vi "Dresden R2R Sputter 03.02.2018 IY24.vi"() -> ()   [LabVIEW 2009] (continued)
                    n17084 = local read "Semi"() -> (w25564:bool)
                    n17085 = case shown="False" w25564 {
                      frame #0 {
                        n17086 = stacked-sequence {
                          frame #0 {
                            n17087 = local read "Semi"() -> (w25565:bool)
                            n17088 = case shown="False" w25565 {
                              frame #0 {
                                n17089 = while {
                                i -> [w25572]
                                stop <- w25568 stop-if-true
                                n17090 = Greater?(x=w25572, y=50) -> (0:w25566:bool)
                                n17091 = case shown="True" w25566 {
                                frame #0 {
                                }
                                frame #1 {
                                n17092 = local write "Error Message"("Start up process cancelled because\nthere is no enough air pressure.\nPlease check air pressure connections." ("Error Message")) -> ()
                                n17093 = local write "Semi"(TRUE ("Semi")) -> ()
                                }
                                }
                                n17094 = local read "Ch2_Air_press_di"() -> (w25567:bool)
                                n17095 = case shown="True" w25567 {
                                tunnel: [TRUE FALSE] -> w25570
                                frame #0 {
                                }
                                frame #1 {
                                n17096 = Wait Until Next ms Multiple(millisecond multiple=u32 200) -> ()  [unwired: 1 out]
                                }
                                }
                                n17097 = local read "Semi"() -> (w25569:bool)
                                n17098 = Or(x=w25570, y=w25569) -> (x .or. y?=w25568:bool)
                                }
                              }
                              frame #1 {
                              }
                            }
                          }
                          frame #1 {
                            n17099 = local read "Semi"() -> (w25578:bool)
                            n17100 = case shown="False" w25578 {
                              frame #0 {
                                n17101 = Wait Until Next ms Multiple(millisecond multiple=u32 1000) -> ()  [unwired: 1 out]
                                n17102 = local write "Ch2_PV0"(TRUE ("PA0")) -> ()
                                n17103 = local write "Ch2_PA0"(TRUE ("PA0")) -> ()
                              }
                              frame #1 {
                              }
                            }
                          }
                        }
                      }
                      frame #1 {
                      }
                    }
                  }
                  frame #2 {
                    n17104 = local read "Semi"() -> (w25582:bool)
                    n17105 = case shown="False" w25582 {
                      frame #0 {
                        n17106 = stacked-sequence {
                          frame #0 {
                            n17107 = local read "Semi"() -> (w25583:bool)
                            n17108 = case shown="False" w25583 {
                              frame #0 {
                                n17109 = while {
                                i -> [w25590]
                                stop <- w25586 stop-if-true
                                n17110 = Greater?(x=w25590, y=50) -> (0:w25584:bool)
                                n17111 = case shown="True" w25584 {
                                frame #0 {
                                }
                                frame #1 {
                                n17112 = local write "Error Message"("Start up process cancelled because\nchamber door is open.\nPlease close the door." ("Error Message")) -> ()
                                n17113 = local write "Semi"(TRUE ("Semi")) -> ()
                                }
                                }
                                n17114 = local read "Ch2_Ds_di"() -> (w25585:bool)
                                n17115 = case shown="True" w25585 {
                                tunnel: [TRUE FALSE] -> w25588
                                frame #0 {
                                }
                                frame #1 {
                                n17116 = Wait Until Next ms Multiple(millisecond multiple=u32 200) -> ()  [unwired: 1 out]
                                }
                                }
                                n17117 = local read "Semi"() -> (w25587:bool)
                                n17118 = Or(x=w25588, y=w25587) -> (x .or. y?=w25586:bool)
                                }
                              }
                              frame #1 {
                              }
                            }
                          }
                          frame #1 {
                            n17119 = local read "Semi"() -> (w25596:bool)
                            n17120 = case shown="False" w25596 {
                              frame #0 {
                                n17121 = local write "Ch2_PV1"(TRUE ("PA0")) -> ()
                                n17122 = local write "Ch2_PA1"(TRUE ("PA0")) -> ()
                                n17123 = Wait Until Next ms Multiple(millisecond multiple=u32 1000) -> ()  [unwired: 1 out]
                              }
                              frame #1 {
                              }
                            }
                          }
                        }
                      }
                      frame #1 {
                      }
                    }
                  }
                  frame #3 {
                    n17124 = local read "Semi"() -> (w25600:bool)
                    n17125 = case shown="False" w25600 {
                      frame #0 {
                        n17126 = stacked-sequence {
                          frame #0 {
                            n17127 = local read "Semi"() -> (w25601:bool)
                            n17128 = case shown="False" w25601 {
                              frame #0 {
                                n17129 = while {
                                i -> [w25608]
                                stop <- w25604 stop-if-true
                                n17130 = Greater?(x=w25608, y=50) -> (0:w25602:bool)
                                n17131 = case shown="True" w25602 {
                                frame #0 {
                                }
                                frame #1 {
                                n17132 = local write "Error Message"("Start up process cancelled because\nsystem water flow is not enough.\nPlease check main water flow connections." ("Error Message")) -> ()
                                n17133 = local write "Semi"(TRUE ("Semi")) -> ()
                                }
                                }
                                n17134 = local read "Cnt_wfs_di"() -> (w25603:bool)
                                n17135 = case shown="False" w25603 {
                                tunnel: [TRUE FALSE] -> w25606
                                frame #0 {
                                }
                                frame #1 {
                                n17136 = Wait Until Next ms Multiple(millisecond multiple=u32 200) -> ()  [unwired: 1 out]
                                }
                                }
                                n17137 = local read "Semi"() -> (w25605:bool)
                                n17138 = Or(x=w25606, y=w25605) -> (x .or. y?=w25604:bool)
                                }
                              }
                              frame #1 {
                              }
                            }
                          }
                          frame #1 {
                            n17139 = local read "Semi"() -> (w25614:bool)
                            n17140 = case shown="False" w25614 {
                              frame #0 {
                                n17141 = Wait Until Next ms Multiple(millisecond multiple=u32 1000) -> ()  [unwired: 1 out]
                                n17142 = local write "Ch2_PV2"(TRUE ("PA0")) -> ()
                                n17143 = local write "Ch2_PA2"(TRUE ("PA0")) -> ()
                              }
                              frame #1 {
                              }
                            }
                          }
                        }
                      }
                      frame #1 {
                      }
                    }
                  }
                  frame #4 {
                    n17144 = local read "Semi"() -> (w25618:bool)
                    n17145 = case shown="False" w25618 {
                      frame #0 {
                        n17146 = disable-structure shown="Disabled" {
                          frame #0 {
                            n17147 = stacked-sequence {
                              frame #0 {
                                n17148 = local read "Semi"() -> (w25619:bool)
                                n17149 = case shown="False" w25619 {
                                frame #0 {
                                n17150 = local write "Ch2_WFC_do"(TRUE ("Ch1_WFC_do")) -> ()
                                }
                                frame #1 {
                                }
                                }
                              }
                              frame #1 {
                                n17151 = local read "Semi"() -> (w25621:bool)
                                n17152 = case shown="False" w25621 {
                                frame #0 {
                                n17153 = while {
                                i -> [w25628]
                                stop <- w25624 stop-if-true
                                n17154 = Greater?(x=w25628, y=50) -> (0:w25622:bool)
                                n17155 = case shown="True" w25622 {
                                frame #0 {
                                }
                                frame #1 {
                                n17156 = local write "Error Message"("Start up process cancelled because\nchamber water flow is not enough.\nPlease check chamber water \nflow connections." ("Error Message")) -> ()
                                n17157 = local write "Semi"(TRUE ("Semi")) -> ()
                                }
                                }
                                n17158 = local read "Ch2_WFS_di"() -> (w25623:bool)
                                n17159 = case shown="False" w25623 {
                                tunnel: [TRUE FALSE] -> w25626
                                frame #0 {
                                }
                                frame #1 {
                                n17160 = Wait Until Next ms Multiple(millisecond multiple=u32 200) -> ()  [unwired: 1 out]
                                n17161 = local write "Ch2_WFC_do"(TRUE ("Ch1_WFC_do")) -> ()
                                }
                                }
                                n17162 = local read "Semi"() -> (w25625:bool)
                                n17163 = Or(x=w25626, y=w25625) -> (x .or. y?=w25624:bool)
                                }
                                }
                                frame #1 {
                                }
                                }
                              }
                              frame #2 {
                                n17164 = local read "Semi"() -> (w25635:bool)
                                n17165 = case shown="False" w25635 {
                                frame #0 {
                                n17166 = Wait Until Next ms Multiple(millisecond multiple=u32 1000) -> ()  [unwired: 1 out]
                                }
                                frame #1 {
                                }
                                }
                              }
                            }
                          }
                          frame #1 {
                          }
                        }
                      }
                      frame #1 {
                      }
                    }
                  }
                  frame #5 {
                    # "ch1 and ch2 trns gv close check"
                    n17167 = local read "Semi"() -> (w25637:bool)
                    n17168 = case shown="False" w25637 {
                      frame #0 {
                        n17169 = stacked-sequence {
                          frame #0 {
                            # "Her ikiside false olduğunda sinyal alnmaz"
                            n17170 = local read "Semi"() -> (w25638:bool)
                            n17171 = case shown="False" w25638 {
                              frame #0 {
                                n17172 = local write "Ch1_Trns_gv_close_do"(TRUE ("Ch1_WFC_do")) -> ()
                              }
                              frame #1 {
                              }
                            }
                          }
                          frame #1 {
                            n17173 = local read "Semi"() -> (w25640:bool)
                            n17174 = case shown="False" w25640 {
                              frame #0 {
                                n17175 = while {
                                i -> [w25647]
                                stop <- w25643 stop-if-true
                                n17176 = Greater?(x=w25647, y=300) -> (0:w25641:bool)
                                n17177 = case shown="True" w25641 {
                                frame #0 {
                                }
                                frame #1 {
                                n17178 = local write "Error Message"("Start up process cancelled because\nchamber Trns GV between \nCH1 and CH2 not closed.\nPlease check  GV connection." ("Error Message")) -> ()
                                n17179 = local write "Semi"(TRUE ("Semi")) -> ()
                                }
                                }
                                n17180 = local read "Ch1_Trns_gv_close_di"() -> (w25642:bool)
                                n17181 = case shown="False" w25642 {
                                tunnel: [TRUE FALSE] -> w25645
                                frame #0 {
                                }
                                frame #1 {
                                n17182 = Wait Until Next ms Multiple(millisecond multiple=u32 200) -> ()  [unwired: 1 out]
                                n17183 = local write "Ch1_Trns_gv_open_do"(FALSE ("Ch1_Trns_gv_open_do")) -> ()
                                n17184 = local write "Ch1_Trns_gv_close_do"(TRUE ("Ch1_Trns_gv_close_do")) -> ()
                                }
                                }
                                n17185 = local read "Semi"() -> (w25644:bool)
                                n17186 = Or(x=w25645, y=w25644) -> (x .or. y?=w25643:bool)
                                }
                              }
                              frame #1 {
                              }
                            }
                          }
                          frame #2 {
                            n17187 = local read "Semi"() -> (w25655:bool)
                            n17188 = case shown="False" w25655 {
                              frame #0 {
                                n17189 = Wait Until Next ms Multiple(millisecond multiple=u32 1000) -> ()  [unwired: 1 out]
                                n17190 = local write "Ch2_PV4"(TRUE ("PA0")) -> ()
                                n17191 = local write "Ch2_PA4"(TRUE ("PA0")) -> ()
                              }
                              frame #1 {
                              }
                            }
                          }
                        }
                      }
                      frame #1 {
                      }
                    }
                  }
                  frame #6 {
                    # "ch2 and ch3 trns gv close check"
                    n17192 = local read "Semi"() -> (w25659:bool)
                    n17193 = case shown="False" w25659 {
                      frame #0 {
                        n17194 = stacked-sequence {
                          frame #0 {
                            # "Her ikiside false olduğunda sinyal alnmaz"
                            n17195 = local read "Semi"() -> (w25660:bool)
                            n17196 = case shown="False" w25660 {
                              frame #0 {
                                n17197 = local write "Ch2_Trns_gv_close_do"(TRUE ("Ch1_WFC_do")) -> ()
                              }
                              frame #1 {
                              }
                            }
                          }
                          frame #1 {
                            n17198 = local read "Semi"() -> (w25662:bool)
                            n17199 = case shown="False" w25662 {
                              frame #0 {
                                n17200 = while {
                                i -> [w25669]
                                stop <- w25665 stop-if-true
                                n17201 = Greater?(x=w25669, y=300) -> (0:w25663:bool)
                                n17202 = case shown="True" w25663 {
                                frame #0 {
                                }
                                frame #1 {
                                n17203 = local write "Error Message"("Start up process cancelled because\nchamber Trns GV between \nCH2 and CH3 not closed.\nPlease check  GV connection." ("Error Message")) -> ()
                                n17204 = local write "Semi"(TRUE ("Semi")) -> ()
                                }
                                }
                                n17205 = local read "Ch2_Trns_gv_close_di"() -> (w25664:bool)
                                n17206 = case shown="False" w25664 {
                                tunnel: [TRUE FALSE] -> w25667
                                frame #0 {
                                }
                                frame #1 {
                                n17207 = Wait Until Next ms Multiple(millisecond multiple=u32 200) -> ()  [unwired: 1 out]
                                n17208 = local write "Ch2_Trns_gv_open_do"(FALSE ("Ch1_Trns_gv_open_do")) -> ()
                                n17209 = local write "Ch2_Trns_gv_close_do"(TRUE ("Ch1_Trns_gv_close_do")) -> ()
                                }
                                }
                                n17210 = local read "Semi"() -> (w25666:bool)
                                n17211 = Or(x=w25667, y=w25666) -> (x .or. y?=w25665:bool)
                                }
                              }
                              frame #1 {
                              }
                            }
                          }
                          frame #2 {
                            n17212 = local read "Semi"() -> (w25677:bool)
                            n17213 = case shown="False" w25677 {
                              frame #0 {
                                n17214 = Wait Until Next ms Multiple(millisecond multiple=u32 1000) -> ()  [unwired: 1 out]
                                n17215 = local write "Ch2_PV5"(TRUE ("PA0")) -> ()
                                n17216 = local write "Ch2_PA5"(TRUE ("PA0")) -> ()
                              }
                              frame #1 {
                              }
                            }
                          }
                        }
                      }
                      frame #1 {
                      }
                    }
                  }
                }
              }
              frame #1 {
              }
            }
          }
          frame #1 {
            # "ROUTINE CHECK"
            n17217 = local read "Semi"() -> (w25681:bool)
            n17218 = case shown="False" w25681 {
              frame #0 {
                n17219 = local read "Ch2_pressure"() -> (w25683:dbl)
                n17220 = Greater Or Equal?(x=w25683, y=0.9) -> (x >= y?=w25682:bool)
                n17221 = case shown="True" w25682 {
                  frame #0 {
                    # "PUMPING CH2 LOWER THAN 0.9 TORR"
                    n17222 = local read "Semi"() -> (w25685:bool)
                    n17223 = case shown="False" w25685 {
                      frame #0 {
                        n17224 = stacked-sequence {
                          frame #0 {
                            # "Close CH-VBV"
                            n17225 = local read "Semi"() -> (w25686:bool)
                            n17226 = case shown="False" w25686 {
                              frame #0 {
                                n17227 = stacked-sequence {
                                frame #0 {
                                n17228 = local read "Semi"() -> (w25687:bool)
                                n17229 = case shown="False" w25687 {
                                frame #0 {
                                n17230 = while {
                                i -> [w25694]
                                stop <- w25688 stop-if-true
                                n17231 = Greater?(x=w25694, y=50) -> (0:w25692:bool)
                                n17232 = case shown="True" w25692 {
                                frame #0 {
                                }
                                frame #1 {
                                n17233 = local write "Semi"(TRUE ("Semi")) -> ()
                                n17234 = local write "Error Message"("Start up process  cancelled\nbecause  CH-VBV not closed.\nPlease check  CH2-VBV connections." ("Error Message")) -> ()
                                }
                                }
                                n17235 = local read "Ch2_Ch_vbv_di"() -> (w25691:bool)
                                n17236 = case shown="True" w25691 {
                                tunnel: [TRUE FALSE] -> w25690
                                frame #0 {
                                }
                                frame #1 {
                                n17237 = Wait Until Next ms Multiple(millisecond multiple=u32 200) -> ()  [unwired: 1 out]
                                n17238 = local write "Ch2_Ch_vbv_do"(FALSE ("Ch1_Tp_bv_do")) -> ()
                                }
                                }
                                n17239 = local read "Semi"() -> (w25689:bool)
                                n17240 = Or(x=w25690, y=w25689) -> (x .or. y?=w25688:bool)
                                }
                                }
                                frame #1 {
                                }
                                }
                                }
                                frame #1 {
                                n17241 = local read "Semi"() -> (w25701:bool)
                                n17242 = case shown="False" w25701 {
                                frame #0 {
                                n17243 = local write "Ch2_PV6"(TRUE ("P03")) -> ()
                                n17244 = Wait Until Next ms Multiple(millisecond multiple=u32 1000) -> ()  [unwired: 1 out]
                                }
                                frame #1 {
                                }
                                }
                                }
                                }
                              }
                              frame #1 {
                              }
                            }
                          }
                          frame #1 {
                            # "Close PL-VBV"
                            n17245 = local read "Semi"() -> (w25704:bool)
                            n17246 = case shown="False" w25704 {
                              frame #0 {
                                n17247 = stacked-sequence {
                                frame #0 {
                                n17248 = local read "Semi"() -> (w25705:bool)
                                n17249 = case shown="False" w25705 {
                                frame #0 {
                                n17250 = while {
                                i -> [w25712]
                                stop <- w25706 stop-if-true
                                n17251 = Greater?(x=w25712, y=50) -> (0:w25710:bool)
                                n17252 = case shown="True" w25710 {
                                frame #0 {
                                }
                                frame #1 {
                                n17253 = local write "Semi"(TRUE ("Semi")) -> ()
                                n17254 = local write "Error Message"("Start up process  cancelled\nbecause  PL-VBV not closed.\nPlease check PL2-VBV connections." ("Error Message")) -> ()
                                }
                                }
                                n17255 = local read "Ch2_Pl_vbv_di"() -> (w25709:bool)
                                n17256 = case shown="True" w25709 {
                                tunnel: [TRUE FALSE] -> w25708
                                frame #0 {
                                }
                                frame #1 {
                                n17257 = Wait Until Next ms Multiple(millisecond multiple=u32 200) -> ()  [unwired: 1 out]
                                n17258 = local write "Ch2_Pl_vbv_do"(FALSE ("Ch1_Tp_bv_do")) -> ()
                                }
                                }
                                n17259 = local read "Semi"() -> (w25707:bool)
                                n17260 = Or(x=w25708, y=w25707) -> (x .or. y?=w25706:bool)
                                }
                                }
                                frame #1 {
                                }
                                }
                                }
                                frame #1 {
                                n17261 = local read "Semi"() -> (w25719:bool)
                                n17262 = case shown="False" w25719 {
                                frame #0 {
                                n17263 = local write "Ch2_PV7"(TRUE ("P03")) -> ()
                                n17264 = Wait Until Next ms Multiple(millisecond multiple=u32 1000) -> ()  [unwired: 1 out]
                                }
                                frame #1 {
                                }
                                }
                                }
                                }
                              }
                              frame #1 {
                              }
                            }
                          }
                          frame #2 {
                            # "Close CH-ATM"
                            n17265 = local read "Semi"() -> (w25722:bool)
                            n17266 = case shown="False" w25722 {
                              frame #0 {
                                n17267 = stacked-sequence {
                                frame #0 {
                                n17268 = local read "Semi"() -> (w25723:bool)
                                n17269 = case shown="False" w25723 {
                                frame #0 {
                                n17270 = while {
                                i -> [w25730]
                                stop <- w25724 stop-if-true
                                n17271 = Greater?(x=w25730, y=50) -> (0:w25728:bool)
                                n17272 = case shown="True" w25728 {
                                frame #0 {
                                }
                                frame #1 {
                                n17273 = local write "Semi"(TRUE ("Semi")) -> ()
                                n17274 = local write "Error Message"("Start up process  cancelled\nbecause CH-ATM not closed.\nPlease check CH2-ATM connections." ("Error Message")) -> ()
                                }
                                }
                                n17275 = local read "Ch2_Ch_atm_di"() -> (w25727:bool)
                                n17276 = case shown="True" w25727 {
                                tunnel: [TRUE FALSE] -> w25726
                                frame #0 {
                                }
                                frame #1 {
                                n17277 = Wait Until Next ms Multiple(millisecond multiple=u32 200) -> ()  [unwired: 1 out]
                                n17278 = local write "Ch2_Ch_atm_do"(TRUE ("Ch1_Tp_bv_do")) -> ()
                                }
                                }
                                n17279 = local read "Semi"() -> (w25725:bool)
                                n17280 = Or(x=w25726, y=w25725) -> (x .or. y?=w25724:bool)
                                }
                                }
                                frame #1 {
                                }
                                }
                                }
                                frame #1 {
                                n17281 = local read "Semi"() -> (w25737:bool)
                                n17282 = case shown="False" w25737 {
                                frame #0 {
                                n17283 = Wait Until Next ms Multiple(millisecond multiple=u32 1000) -> ()  [unwired: 1 out]
                                n17284 = local write "Ch2_PV8"(TRUE ("P03")) -> ()
                                }
                                frame #1 {
                                }
                                }
                                }
                                }
                              }
                              frame #1 {
                              }
                            }
                          }
                          frame #3 {
                            # "Close PL-ATM"
                            n17285 = local read "Semi"() -> (w25740:bool)
                            n17286 = case shown="False" w25740 {
                              frame #0 {
                                n17287 = stacked-sequence {
                                frame #0 {
                                n17288 = local read "Semi"() -> (w25741:bool)
                                n17289 = case shown="False" w25741 {
                                frame #0 {
                                n17290 = while {
                                i -> [w25748]
                                stop <- w25742 stop-if-true
                                n17291 = Greater?(x=w25748, y=50) -> (0:w25746:bool)
                                n17292 = case shown="True" w25746 {
                                frame #0 {
                                }
                                frame #1 {
                                n17293 = local write "Semi"(TRUE ("Semi")) -> ()
                                n17294 = local write "Error Message"("Start up process  cancelled\nbecause PL-ATM not closed.\nPlease check PL2-ATM connections." ("Error Message")) -> ()
                                }
                                }
                                n17295 = local read "Ch2_Pl_atm_di"() -> (w25745:bool)
                                n17296 = case shown="True" w25745 {
                                tunnel: [TRUE FALSE] -> w25744
                                frame #0 {
                                }
                                frame #1 {
                                n17297 = Wait Until Next ms Multiple(millisecond multiple=u32 200) -> ()  [unwired: 1 out]
                                n17298 = local write "Ch2_Pl_atm_do"(TRUE ("Ch1_Tp_bv_do")) -> ()
                                }
                                }
                                n17299 = local read "Semi"() -> (w25743:bool)
                                n17300 = Or(x=w25744, y=w25743) -> (x .or. y?=w25742:bool)
                                }
                                }
                                frame #1 {
                                }
                                }
                                }
                                frame #1 {
                                n17301 = local read "Semi"() -> (w25755:bool)
                                n17302 = case shown="False" w25755 {
                                frame #0 {
                                n17303 = local write "Ch2_PV9"(TRUE ("P03")) -> ()
                                n17304 = Wait Until Next ms Multiple(millisecond multiple=u32 1000) -> ()  [unwired: 1 out]
                                }
                                frame #1 {
                                }
                                }
                                }
                                }
                              }
                              frame #1 {
                              }
                            }
                          }
                          frame #4 {
                            # "START MP"
                            n17305 = local read "Semi"() -> (w25758:bool)
                            n17306 = case shown="False" w25758 {
                              frame #0 {
                                n17307 = stacked-sequence {
                                frame #0 {
                                n17308 = local read "Semi"() -> (w25759:bool)
                                n17309 = case shown="False" w25759 {
                                frame #0 {
                                n17310 = while {
                                i -> [w25766]
                                stop <- w25760 stop-if-true
                                n17311 = Greater?(x=w25766, y=50) -> (0:w25764:bool)
                                n17312 = case shown="True" w25764 {
                                frame #0 {
                                }
                                frame #1 {
                                n17313 = local write "Semi"(TRUE ("Semi")) -> ()
                                n17314 = local write "Error Message"("Start up process  cancelled\nbecause MP not started.\nPlease check MP2 connections." ("Error Message")) -> ()
                                }
                                }
                                n17315 = local read "Ch2_Mp_di"() -> (w25763:bool)
                                n17316 = case shown="False" w25763 {
                                tunnel: [FALSE TRUE] -> w25762
                                frame #0 {
                                n17317 = Wait Until Next ms Multiple(millisecond multiple=u32 200) -> ()  [unwired: 1 out]
                                n17318 = local write "Ch2_Mp_do"(TRUE ("Ch1_Tp_bv_do")) -> ()
                                }
                                frame #1 {
                                }
                                }
                                n17319 = local read "Semi"() -> (w25761:bool)
                                n17320 = Or(x=w25762, y=w25761) -> (x .or. y?=w25760:bool)
                                }
                                }
                                frame #1 {
                                }
                                }
                                }
                                frame #1 {
                                n17321 = local read "Semi"() -> (w25773:bool)
                                n17322 = case shown="False" w25773 {
                                frame #0 {
                                n17323 = local write "Ch2_PV10"(TRUE ("P03")) -> ()
                                n17324 = Wait Until Next ms Multiple(millisecond multiple=u32 1000) -> ()  [unwired: 1 out]
                                }
                                frame #1 {
                                }
                                }
                                }
                                }
                              }
                              frame #1 {
                              }
                            }
                          }
                          frame #5 {
                            # "CHECK PL-PRESSURE"
                            n17325 = local read "Semi"() -> (w25776:bool)
                            n17326 = case shown="False" w25776 {
                              frame #0 {
                                n17327 = stacked-sequence {
                                frame #0 {
                                n17328 = local read "Semi"() -> (w25777:bool)
                                n17329 = case shown="False" w25777 {
                                frame #0 {
                                n17330 = while {
                                i -> [w25786]
                                stop <- w25781 stop-if-true
                                n17331 = Greater?(x=w25786, y=240) -> (0:w25784:bool)
                                n17332 = case shown="True" w25784 {
                                frame #0 {
                                }
                                frame #1 {
                                n17333 = local write "Semi"(TRUE ("Semi")) -> ()
                                n17334 = local write "Error Message"("Start up process was cancelled.\nPlease check Pipeline \nvacuum connections." ("Error Message")) -> ()
                                }
                                }
                                n17335 = local read "Pl_pg_press_ch2"() -> (w25780:dbl)
                                n17336 = Less?(x=w25780, y=0.9) -> (x < y?=w25778:bool)
                                n17337 = case shown="False" w25778 {
                                tunnel: [FALSE TRUE] -> w25783
                                frame #0 {
                                n17338 = Wait Until Next ms Multiple(millisecond multiple=u32 200) -> ()  [unwired: 1 out]
                                }
                                frame #1 {
                                }
                                }
                                n17339 = local read "Semi"() -> (w25782:bool)
                                n17340 = Or(x=w25783, y=w25782) -> (x .or. y?=w25781:bool)
                                }
                                }
                                frame #1 {
                                }
                                }
                                }
                                frame #1 {
                                n17341 = local read "Semi"() -> (w25792:bool)
                                n17342 = case shown="False" w25792 {
                                frame #0 {
                                n17343 = local write "Ch2_PV11"(TRUE ("P03")) -> ()
                                n17344 = Wait Until Next ms Multiple(millisecond multiple=u32 1000) -> ()  [unwired: 1 out]
                                }
                                frame #1 {
                                }
                                }
                                }
                                }
                              }
                              frame #1 {
                              }
                            }
                          }
                          frame #6 {
                            # "CHECK CH-PRESSURE"
                            n17345 = local read "Semi"() -> (w25795:bool)
                            n17346 = case shown="False" w25795 {
                              frame #0 {
                                n17347 = stacked-sequence {
                                frame #0 {
                                n17348 = local read "Semi"() -> (w25796:bool)
                                n17349 = case shown="False" w25796 {
                                frame #0 {
                                n17350 = while {
                                i -> [w25805]
                                stop <- w25800 stop-if-true
                                n17351 = Greater?(x=w25805, y=50) -> (0:w25803:bool)
                                n17352 = case shown="True" w25803 {
                                frame #0 {
                                }
                                frame #1 {
                                n17353 = local write "Semi"(TRUE ("Semi")) -> ()
                                n17354 = local write "Error Message"("Start up process was cancelled.\nPlease check chamber \nvacuum connections." ("Error Message")) -> ()
                                }
                                }
                                n17355 = local read "Ch2_pressure"() -> (w25799:dbl)
                                n17356 = Less?(x=w25799, y=0.9) -> (x < y?=w25797:bool)
                                n17357 = case shown="False" w25797 {
                                tunnel: [FALSE TRUE] -> w25802
                                frame #0 {
                                n17358 = Wait Until Next ms Multiple(millisecond multiple=u32 200) -> ()  [unwired: 1 out]
                                }
                                frame #1 {
                                }
                                }
                                n17359 = local read "Semi"() -> (w25801:bool)
                                n17360 = Or(x=w25802, y=w25801) -> (x .or. y?=w25800:bool)
                                }
                                }
                                frame #1 {
                                }
                                }
                                }
                                frame #1 {
                                n17361 = local read "Semi"() -> (w25811:bool)
                                n17362 = case shown="False" w25811 {
                                frame #0 {
                                n17363 = local write "Ch2_PV12"(TRUE ("P03")) -> ()
                                n17364 = Wait Until Next ms Multiple(millisecond multiple=u32 1000) -> ()  [unwired: 1 out]
                                }
                                frame #1 {
                                }
                                }
                                }
                                }
                              }
                              frame #1 {
                              }
                            }
                          }
                          frame #7 {
                            # "OPEN TP-BV"
                            n17365 = local read "Semi"() -> (w25814:bool)
                            n17366 = case shown="False" w25814 {
                              frame #0 {
                                n17367 = stacked-sequence {
                                frame #0 {
                                n17368 = local read "Semi"() -> (w25815:bool)
                                n17369 = case shown="False" w25815 {
                                frame #0 {
                                n17370 = while {
                                i -> [w25822]
                                stop <- w25817 stop-if-true
                                n17371 = Greater?(x=w25822, y=50) -> (0:w25820:bool)
                                n17372 = case shown="True" w25820 {
                                frame #0 {
                                }
                                frame #1 {
                                n17373 = local write "Semi"(TRUE ("Semi")) -> ()
                                n17374 = local write "Error Message"("Start up process  cancelled\nbecause  TP-BV not opened.\nPlease check TP-BV2 connections." ("Error Message")) -> ()
                                }
                                }
                                n17375 = local read "Ch2_Tp_bv_di"() -> (w25816:bool)
                                n17376 = case shown="False" w25816 {
                                tunnel: [FALSE TRUE] -> w25819
                                frame #0 {
                                n17377 = Wait Until Next ms Multiple(millisecond multiple=u32 200) -> ()  [unwired: 1 out]
                                n17378 = local write "Ch2_Tp_bv_do"(TRUE ("Ch1_Tp_bv_do")) -> ()
                                }
                                frame #1 {
                                }
                                }
                                n17379 = local read "Semi"() -> (w25818:bool)
                                n17380 = Or(x=w25819, y=w25818) -> (x .or. y?=w25817:bool)
                                }
                                }
                                frame #1 {
                                }